vi "UHR-Fleezers Control (host) - 10.2.vi"() -> ()   [LabVIEW 2009] (continued)
                n756 = Build Array (concatenate)(w3470, w3469, w3463) -> (w3468:dbl[])
              }
              frame #1 {
                w3484 = 0.0 ("f")
                w3481 = FALSE ("Save APD Data\nwith Trap Data")
                # "calibration"
                n757 = Boolean To (0,1)(Boolean=w3481) -> (0, 1=w3486:i16)
                n758 = To Double Precision Float(number=w3486) -> (double precision float=w3485:dbl)
                n759 = Build Array(w3485, w3484, w3484, w3484, w3484) -> (w3483:dbl[])
                n760 = Build Array(w3482, w3487, w3487, w3494, w3493, 1.0 ("t")) -> (w3491:dbl[])
                n761 = Build Array (concatenate)(w3491, w3490, w3483) -> (w3489:dbl[])
                "Calibrating Trap..." <- TRUE ("Calibrating...")
              }
              frame #2 {
                w3501 = 0.0 ("f")
                # "scan dir (x/y = 0/1)"
                # "cycles/step"
                # "n scans (f/b)"
                # "steps"
                # "freq. range"
                # "AOD raster scan"
                n762 = local read "Number of F/B Scans (AOD)"() -> (w3508:u16)
                n763 = local read "Cycles/step (AOD)"() -> (w3510:u64)
                n764 = local read "Scan Range (MHz)"() -> (w3513:dbl)
                n765 = local read "Scan steps (AOD)"() -> (w3512:u64)
                n766 = local read "Scan BD"() -> (w3520:bool)
                n767 = local read "Save ave N"() -> (w3525:dbl)
                n768 = Boolean To (0,1)(Boolean=w3520) -> (0, 1=w3519:i16)
                n769 = To Double Precision Float(number=w3508) -> (double precision float=w3507:dbl)
                n770 = To Double Precision Float(number=w3512) -> (double precision float=w3511:dbl)
                n771 = To Double Precision Float(number=w3510) -> (double precision float=w3509:dbl)
                n772 = To Double Precision Float(number=w3519) -> (double precision float=w3518:dbl)
                n773 = Multiply(x=w3525, y=w3503) -> (x*y=w3524:dbl)
                n774 = To Double Precision Float(number=w3496) -> (double precision float=w3502:dbl)
                n775 = Build Array(w3502, w3501, w3501, w3501, w3501) -> (w3499:dbl[])
                n776 = local read "N sets should be saved"() -> (w3505:dbl)
                n777 = Build Array(w3518, w3513, w3511, w3509, w3507) -> (w3515:dbl[])
                n778 = Build Array(w3498, w3503, w3524, w3523, w3522, 2.0 ("t")) -> (w3517:dbl[])
                n779 = Round Toward +Infinity(x=w3505) -> (ceil(x): smallest int >= x=w3506:dbl)
                n780 = Build Array (concatenate)(w3517, w3516, w3499, w3515) -> (w3514:dbl[])
                n781 = To Unsigned Long Integer(number=w3506) -> (unsigned 32bit integer=w3504:u32)
              }
              frame #3 {
                w3534 = 0.0 ("f")
                # "MCL raster scan"
                n782 = local read "Number of scans (MCL)"() -> (w3529:u64)
                n783 = local read "Scan lines (y)"() -> (w3528:u64)
                n784 = local read "2D or 1D Scan"() -> (w3531:bool)
                n785 = local read "Scan Range (V)\n(of steps)"() -> (w3550:dbl)
                n786 = local read "Fast Scan Dir"() -> (w3557:bool)
                n787 = local read "Cycles/step (MCL)"() -> (w3547:u64)
                n788 = local read "Scan steps (MCL)"() -> (w3549:u64)
                n789 = Select(t=w3528, s=w3531, f=w3529) -> (s? t:f=w3530:u64)
                n790 = Boolean To (0,1)(Boolean=w3531) -> (0, 1=w3533:i16)
                n791 = local read "Save ave N"() -> (w3562:dbl)
                n792 = local read "Initial X"() -> (w3536:dbl)
                n793 = local read "Initial Y"() -> (w3535:dbl)
                n794 = To Double Precision Float(number=w3533) -> (double precision float=w3532:dbl)
                n795 = Boolean To (0,1)(Boolean=w3557) -> (0, 1=w3556:i16)
                n796 = To Double Precision Float(number=w3530) -> (double precision float=w3545:dbl)
                n797 = To Double Precision Float(number=w3549) -> (double precision float=w3548:dbl)
                n798 = To Double Precision Float(number=w3547) -> (double precision float=w3546:dbl)
                n799 = To Double Precision Float(number=w3556) -> (double precision float=w3555:dbl)
                n800 = Multiply(x=w3562, y=w3541) -> (x*y=w3561:dbl)
                n801 = To Double Precision Float(number=w3526) -> (double precision float=w3540:dbl)
                n802 = local read "N sets should be saved (MCL)"() -> (w3543:dbl)
                n803 = Build Array(w3540, w3532, w3534, w3534, w3534) -> (w3538:dbl[])
                n804 = Build Array(w3555, w3550, w3548, w3546, w3545, w3536, w3535) -> (w3552:dbl[])
                n805 = Build Array(w3537, w3541, w3561, w3560, w3559, 3.0 ("t")) -> (w3554:dbl[])
                n806 = Round Toward +Infinity(x=w3543) -> (ceil(x): smallest int >= x=w3544:dbl)
                n807 = Build Array (concatenate)(w3554, w3553, w3538, w3552) -> (w3551:dbl[])
                n808 = To Unsigned Long Integer(number=w3544) -> (unsigned 32bit integer=w3542:u32)
              }
            }
            n809 = local read "Index"() -> (w3401:dbl)
            n810 = call "Create new save file.vi"("Insert"="", "Ext"=".dat", "Index In"=w3401) -> ("Path Out"=w3360:path, "Index Out"=w3373:dbl)
            n811 = local write "Save file name"(w3360) -> ()
            n812 = local write "Index"(w3373) -> ()
            n813 = local write "Save index"(w3373) -> ()
            n814 = Array Size(array=w3384) -> (size(s)=w3385:i32)
            n815 = Open/Create/Replace File(file path (use dialog)=w3360, operation (0:open)=T33."create", access (0:read/write)=enum16{"read/write", "read-only", "write-only"}."write-only") -> (refnum out=w3398:refnum<file>)  [unwired: 1 in, 4 out]
            n816 = local write "Saving..."(TRUE ("Saving...")) -> ()
            n817 = To Double Precision Float(number=w3385) -> (double precision float=w3383:dbl)
            n818 = String Length(string="Comment (data description)") -> (length=w3381:i32)
            n819 = To Double Precision Float(number=w3381) -> (double precision float=w3380:dbl)
            n820 = Deny Access(7:w3398) -> (3:w3397:refnum<file>)  [unwired: 1 in, 2 out]
            n821 = Build Array (concatenate)(w3383, w3384, w3380) -> (w3382:dbl[])
            n822 = case shown="True" w3358 {
              tunnel: w3360 -> [_ w3412]
              tunnel: [refnum<k0> refnum w3411] -> w3359
              frame #0 {
              }
              frame #1 {
                w3407 = 0.0 ("element")
                n823 = Path To String(path=w3412) -> (string=w3426:string)
                n824 = Build Array(w3407, w3407, w3407, w3407, w3407, w3407, w3407, w3407) -> (w3408:dbl[])
                n825 = String Length(string=w3426) -> (length=w3425:i32)
                n826 = Subtract(x=w3425, y=4) -> (x-y=w3423:i32)
                n827 = Array Size(array=w3408) -> (size(s)=w3410:i32)
                n828 = String Subset(string=w3426, length (rest)=w3423) -> (substring=w3422:string)  [unwired: 1 out]
                n829 = To Double Precision Float(number=w3410) -> (double precision float=w3409:dbl)
                n830 = Concatenate Strings(w3422, "_pos.dat" ("string")) -> (w3420:string)
                n831 = Build Array (concatenate)(w3409, w3408) -> (w3406:dbl[])
                n832 = String To Path(string=w3420) -> (path=w3416:path)
                n833 = Open/Create/Replace File(file path (use dialog)=w3416, operation (0:open)=T33."create", access (0:read/write)=enum16{"read/write", "read-only", "write-only"}."write-only") -> (refnum out=w3417:refnum<file>)  [unwired: 1 in, 4 out]
                n834 = Deny Access(7:w3417) -> (3:w3413:refnum<file>)  [unwired: 1 in, 2 out]
                n835 = Write to Binary File(file (use dialog)=w3413, data=w3406, 5:FALSE ("prepend array or string size? (T)"), 9:T34."big-endian, network order" ("byte order (0:big-endian, network order)")) -> (refnum out=w3411:refnum<file>)  [unwired: 1 in, 3 out]
              }
            }
            n836 = case "If fluorescence data to be saved" shown="True" w3371 {
              tunnel: w3360 -> [_ w3450]
              tunnel: [refnum<k0> refnum w3430] -> w3372
              frame #0 {
              }
              frame #1 {
                w3429 = 0.0
                n837 = local read "APD Integration Time (s)"() -> (w3435:dbl)
                n838 = local read "N APD Samp/step"() -> (w3428:dbl)
                n839 = Path To String(path=w3450) -> (string=w3449:string)
                n840 = String Length(string=w3449) -> (length=w3448:i32)
                n841 = Subtract(x=w3448, y=4) -> (x-y=w3446:i32)
                n842 = String Subset(string=w3449, length (rest)=w3446) -> (substring=w3445:string)  [unwired: 1 out]
                n843 = Build Array(w3435, w3428, w3429, w3429, w3429, w3429, w3429, w3429) -> (w3432:dbl[])
                n844 = Concatenate Strings(w3445, "_fl.dat" ("string")) -> (w3443:string)
                n845 = Array Size(array=w3432) -> (size(s)=w3434:i32)
                n846 = String To Path(string=w3443) -> (path=w3439:path)
                n847 = Open/Create/Replace File(file path (use dialog)=w3439, operation (0:open)=T33."create", access (0:read/write)=enum16{"read/write", "read-only", "write-only"}."write-only") -> (refnum out=w3440:refnum<file>)  [unwired: 1 in, 4 out]
                n848 = Deny Access(7:w3440) -> (3:w3436:refnum<file>)  [unwired: 1 in, 2 out]
                n849 = To Double Precision Float(number=w3434) -> (double precision float=w3433:dbl)
                n850 = Build Array (concatenate)(w3433, w3432) -> (w3431:dbl[])
                n851 = Write to Binary File(file (use dialog)=w3436, data=w3431, 5:FALSE ("prepend array or string size? (T)"), 9:T34."big-endian, network order" ("byte order (0:big-endian, network order)")) -> (refnum out=w3430:refnum<file>)  [unwired: 1 in, 3 out]
              }
            }
            n852 = Write to Binary File(file (use dialog)=w3397, data=w3382, 5:w3378, 9:w3376) -> (refnum out=w3379:refnum<file>)  [unwired: 1 in, 3 out]
            n853 = Write to Binary File(file (use dialog)=w3379, data="Comment (data description)", 5:w3378, 9:w3376) -> (refnum out=w3375:refnum<file>)  [unwired: 1 in, 3 out]
          }
        }
      }
      frame #1 {
        n854 = local read "Saving..."() -> (w3575:bool)
        n855 = case shown="True" w3575 {
          tunnel: w3579 -> [_ w3589]
          tunnel: w3578 -> [_ w3603]
          tunnel: w3577 -> [_ w3599]
          tunnel: w3576 -> [_ w3598]
          tunnel: w3574 -> [_ w3597]
          tunnel: w3573 -> [_ w3592]
          tunnel: w3572 -> [_ w3591]
          tunnel: w3571 -> [_ w3590]
          tunnel: w3570 -> [_ w3588]
          tunnel: w3569 -> [_ w3586]
          tunnel: w3568 -> [_ w3585]
          tunnel: w3567 -> [_ w3584]
          tunnel: w3566 -> [_ w3583]
          tunnel: w3565 -> [_ w3582]
          tunnel: w3564 -> [_ w3581]
          tunnel: w3563 -> [_ w3580]
          frame #0 {
          }
          frame #1 {
            n856 = Multiply(x=w3589, y=w3588) -> (x*y=→"Time (s)":dbl)
            n857 = Less Or Equal?(x=w3589, y=w3597) -> (x <= y?=w3601:bool)
            n858 = Or(x="Stop Saving", y="Abort save 2") -> (x .or. y?=w3593:bool)
            n859 = Not(x=w3593) -> (.not. x?=w3602:bool)
            n860 = And(x=w3601, y=w3602) -> (x .and. y?=w3600:bool)
            n861 = case shown="True" w3600 {
              tunnel: w3603 -> [w3610 w3678]
              tunnel: [0.0 w3681] -> w3596
              tunnel: w3589 -> [_ w3679]
              tunnel: w3597 -> [_ w3680]
              tunnel: w3599 -> [_ w3675]
              tunnel: w3598 -> [_ _]
              tunnel: w3592 -> [w3608 w3668]
              tunnel: w3591 -> [w3607 w3669]
              tunnel: w3590 -> [_ w3667]
              tunnel: w3586 -> [_ w3666]
              tunnel: w3585 -> [_ w3620]
              tunnel: w3584 -> [_ w3659]
              tunnel: w3583 -> [_ w3637]
              tunnel: w3582 -> [w3604 w3618]
              tunnel: w3581 -> [w3605 w3617]
              tunnel: w3580 -> [_ w3614]
              frame #0 {
                w3606 = FALSE
                n862 = Close File(refnum=w3610) -> ()  [unwired: 1 in, 2 out]
                n863 = case shown="True" w3607 {
                  tunnel: w3608 -> [_ w3612]
                  frame #0 {
                  }
                  frame #1 {
                    n864 = Close File(refnum=w3612) -> ()  [unwired: 1 in, 2 out]
                  }
                }
                n865 = case shown="True" w3604 {
                  tunnel: w3605 -> [_ w3611]
                  frame #0 {
                  }
                  frame #1 {
                    n866 = Close File(refnum=w3611) -> ()  [unwired: 1 in, 2 out]
                  }
                }
                n867 = local write "Raster Scanning..."(w3606) -> ()
                n868 = local write "Calibrating Trap..."(w3606) -> ()
                n869 = call <vilib>:"Beep.vi"() -> ()  [unwired: 3 in, 9 out]
                n870 = local write "Stop Saving"(w3606) -> ()
                "Saving..." <- w3606
              }
              frame #1 {
                n871 = local read "Calibrating Trap..."() -> (w3670:bool)
                n872 = case "Write fl. data" shown="True" w3669 {
                  tunnel: w3668 -> [_ w3704]
                  tunnel: w3667 -> [_ w3703]
                  frame #0 {
                  }
                  frame #1 {
                    n873 = Write to Binary File(file (use dialog)=w3704, data=w3703, 5:FALSE ("prepend array or string size? (T)"), 9:T34."big-endian, network order" ("byte order (0:big-endian, network order)")) -> ()  [unwired: 1 in, 4 out]
                  }
                }
                n874 = Greater?(x="Save ave N", y=1.0) -> (0:w3673:bool)
                n875 = Not(x=w3670) -> (.not. x?=w3672:bool)
                n876 = And(x=w3672, y=w3673) -> (x .and. y?=w3615:bool)
                n877 = case shown="True" w3615 {
                  tunnel: w3614 -> [w3684 w3695]
                  tunnel: [w3684 w3687] -> w3613
                  tunnel: "Save ave N" -> [_ w3688]
                  frame #0 {
                  }
                  frame #1 {
                    w3685 = 2 ("dimension size")
                    n878 = Array Size(array=w3695) -> (size(s)=w3689:i32)
                    n879 = Divide(x=w3689, y=w3685) -> (x/y=w3693:dbl)
                    n880 = Reshape Array(w3695, w3693, w3685) -> (w3694:u64[][])
                    n881 = Transpose 2D Array(2D array=w3694) -> (transposed array=w3692:u64[][])
                    n882 = for {
                      tunnel: w3692 -> [w3697] mode=indexing
                      tunnel: [w3696] -> w3686 mode=indexing
                      tunnel: w3688 -> [w3698]
                      workers-P: _ -> [_]
                      n883 = call "downsample 1D array - U64.vi"("Ave N"=w3698, "Array In"=w3697) -> ("Array Out"=w3696:u64[])  [unwired: 1 in]
                    }
                    n884 = Transpose 2D Array(2D array=w3686) -> (transposed array=w3691:u64[][])
                    n885 = Divide(x=w3689, y=w3688) -> (x/y=w3690:dbl)
                    n886 = Reshape Array(w3691, w3690) -> (w3687:u64[])
                  }
                }
                n887 = case shown="True" w3615 {
                  tunnel: w3675 -> [w3707 w3719]
                  tunnel: [w3707 w3711] -> w3671
                  tunnel: "Save ave N" -> [_ w3712]
                  tunnel: w3666 -> [_ w3710]
                  frame #0 {
                  }
                  frame #1 {
                    n888 = Array Size(array=w3719) -> (size(s)=w3713:i32)
                    n889 = Array Size(array=w3710) -> (size(s)=w3709:i32)
                    n890 = Divide(x=w3713, y=w3709) -> (x/y=w3717:dbl)
                    n891 = Reshape Array(w3719, w3717, w3709) -> (w3718:i16[][])
                    n892 = Transpose 2D Array(2D array=w3718) -> (transposed array=w3716:i16[][])
                    n893 = for {
                      tunnel: w3716 -> [w3722] mode=indexing
                      tunnel: [w3721] -> w3708 mode=indexing
                      tunnel: w3712 -> [w3720]
                      workers-P: _ -> [_]
                      n894 = call "downsample 1D array - I16.vi"("Ave N"=w3720, "Array In"=w3722) -> ("Array Out"=w3721:i16[])  [unwired: 1 out]
                    }
                    n895 = Transpose 2D Array(2D array=w3708) -> (transposed array=w3715:i16[][])
                    n896 = Divide(x=w3713, y=w3712) -> (x/y=w3714:dbl)
                    n897 = Reshape Array(w3715, w3714) -> (w3711:i16[])
                  }
                }
                n898 = Index Array(array=w3637, index=1) -> (element=w3640:waveform(dbl))
                n899 = Index Array(array=w3637, index=0) -> (element=w3642:waveform(dbl))
                n900 = Unbundle By Name(w3640) -> ("Y"=w3644:dbl[])
                n901 = Unbundle By Name(w3642) -> ("Y"=w3652:dbl[])
                n902 = case "Write trap pos. data" shown="True" w3618 {
                  tunnel: w3617 -> [_ w3700]
                  tunnel: w3613 -> [_ w3699]
                  frame #0 {
                  }
                  frame #1 {
                    n903 = Write to Binary File(file (use dialog)=w3700, data=w3699, 5:FALSE ("prepend array or string size? (T)"), 9:T34."big-endian, network order" ("byte order (0:big-endian, network order)")) -> ()  [unwired: 1 in, 4 out]
                  }
                }
                n904 = Write to Binary File(file (use dialog)=w3678, data=w3671, 5:FALSE ("prepend array or string size? (T)"), 9:T34."big-endian, network order" ("byte order (0:big-endian, network order)")) -> ()  [unwired: 1 in, 4 out]
                n905 = feedback #26(w3644) -> (w3646:dbl[])
                n906 = Build Array (concatenate)(w3646, w3644) -> (w3645:dbl[])
                n907 = Select(t=w3644, s=w3620, f=w3645) -> (s? t:f=w3630:dbl[])
                n908 = feedback #27(w3652) -> (w3665:dbl[])
                n909 = Build Array (concatenate)(w3665, w3652) -> (w3664:dbl[])
                n910 = Select(t=w3652, s=w3620, f=w3664) -> (s? t:f=w3639:dbl[])
                n911 = Divide(x=w3679, y=w3680) -> (x/y=w3682:dbl)
                n912 = Multiply(x=w3682, y=100.0) -> (x*y=w3681:dbl)
                n913 = Build Array(w3639, w3630) -> (→"Saved APD":dbl[][])
                n914 = Array Size(array=w3639) -> (size(s)=w3657:i32)
                n915 = Unbundle By Name(w3659) -> ("Y"=w3663:dbl[])
                n916 = Subtract(x=w3657, y="N pts to average") -> (x-y=w3633:i32)
                n917 = Multiply(x="N pts to average", y=u16 2) -> (x*y=w3634:u16)
                n918 = Subtract(x=w3657, y=w3634) -> (x-y=w3632:i32)
                n919 = feedback #28(w3663) -> (w3662:dbl[])
                n920 = Build Array (concatenate)(w3662, w3663) -> (w3661:dbl[])
                n921 = Select(t=w3663, s=w3620, f=w3661) -> (s? t:f=w3660:dbl[])
                "Trap Delta Graph" <- w3660
                n922 = Array Subset(array=w3639, index=w3633, length="N pts to average") -> (w3656:dbl[])
                n923 = Array Subset(array=w3639, index=w3632, length="N pts to average") -> (w3655:dbl[])
                n924 = Array Subset(array=w3630, index=w3633, length="N pts to average") -> (w3636:dbl[])
                n925 = Array Subset(array=w3630, index=w3632, length="N pts to average") -> (w3635:dbl[])
                n926 = call <vilib>:"Mean.vi"("X"=w3656) -> ("mean"=w3654:dbl)  [unwired: 1 out]
                n927 = call <vilib>:"Mean.vi"("X"=w3636) -> ("mean"=w3629:dbl)  [unwired: 1 out]
                n928 = call <vilib>:"Mean.vi"("X"=w3655) -> ("mean"=w3653:dbl)  [unwired: 1 out]
                n929 = call <vilib>:"Mean.vi"("X"=w3635) -> ("mean"=w3628:dbl)  [unwired: 1 out]
                n930 = Subtract(x=w3629, y=w3628) -> (x-y=w3619:dbl)
                "Delta Fl. 2" <- w3619
                n931 = Subtract(x=w3654, y=w3653) -> (x-y=w3651:dbl)
                "Delta Fl. 1" <- w3651
                n932 = Initialize Array(w3651, 1 ("dimension size")) -> (w3648:dbl[])
                n933 = Initialize Array(w3619, 1 ("dimension size")) -> (w3625:dbl[])
                n934 = feedback #29(w3648) -> (w3649:dbl[])
                n935 = Build Array (concatenate)(w3649, w3648) -> (w3647:dbl[])
                n936 = feedback #30(w3625) -> (w3626:dbl[])
                n937 = Build Array (concatenate)(w3626, w3625) -> (w3624:dbl[])
                n938 = Select(t=w3648, s=w3620, f=w3647) -> (s? t:f=w3623:dbl[])
                n939 = Select(t=w3625, s=w3620, f=w3624) -> (s? t:f=w3622:dbl[])
                n940 = Build Array(w3623, w3622) -> (→"Save APD Deriv":dbl[][])
              }
            }
            "Progress" <- w3596
            "Progress 2" <- w3596
          }
        }
      }
    }
    n941 = Bundle By Name(cluster=w927, "Green FB Ch 0"=w926, "Green FB Ch 1"=w925) -> (w905:T41)
    "Green FB Signals (V)" <- w905
    n942 = Unbundle By Name(w905) -> ("Green FB Ch 2"=→"Green FB Plot":dbl)
    n943 = local read "wait to reset values"() -> (w997:bool)
    n944 = Not(x=w994) -> (.not. x?=w998:bool)
    n945 = And(x=w998, y=w997) -> (x .and. y?=w999:bool)
    n946 = case "Part of MCL raster scanning: returns to initial positions after scan done" shown="True" w999 {
      tunnel: w1002 -> [w2371 w2378]
      tunnel: [w2371 w2377] -> w1001
      tunnel: w996 -> [w2370 w2376]
      tunnel: [w2370 w2375] -> w995
      frame #0 {
      }
      frame #1 {
        w2386 = 10.0 ("y")
        w2385 = 32767.0 ("y")
        # "to return scan values\nafter a synchronous \nAOM scan"
        n947 = local read "AO2"() -> (w2379:dbl)
        n948 = local read "AO1"() -> (w2380:dbl)
        n949 = Multiply(x=w2380, y=w2385) -> (x*y=w2382:dbl)
        n950 = local write "wait to reset values"(FALSE ("wait to reset values")) -> ()
        n951 = Multiply(x=w2379, y=w2385) -> (x*y=w2384:dbl)
        n952 = Divide(x=w2382, y=w2386) -> (x/y=w2381:dbl)
        n953 = Divide(x=w2384, y=w2386) -> (x/y=w2383:dbl)
        n954 = To Word Integer(number=w2381) -> (16bit integer=w2387:i16)
        n955 = To Word Integer(number=w2383) -> (16bit integer=w2388:i16)
        n956 = local read "Total Counts (ticks)"() -> (w2372:u32)
        n957 = xnode "Read/Write Control"("FPGA VI Reference In"=w2378, "error in"=w2376, "AO1"=w2387, "AO2"=w2388, "MCL count"=w2372) -> ("FPGA VI Reference Out"=w2377:T21, "error out"=w2375:errorcluster)
        n958 = local read "Scan Range (V)\n(of steps)"() -> (w2373:dbl)
        n959 = property on="Scan Range (V)\n(of steps)" class="DigNum (strict)"("Val(Sgnl)"=w2373) -> ()  [unwired: 2 in, 2 out]
      }
    }
    n960 = node-c288() -> ()  [unwired: 2 out]
  }
  n961 = disable-structure shown="Disabled" {
    disable-tunnel: [w3796 _] -> w205
    disable-tunnel: w8 -> [w3795 _]
    frame #0 {
      n962 = node-c288() -> (w3798:T23)  [unwired: 4 out]
      n963 = timed-loop "Rough control of MCL mirror stage (debugging)" {
        tunnel: w3795 -> [w3801]
        tunnel: [w3800] -> w3796
        timing: w3798 -> [_]
        timing-out: [_] -> w3797
        stop <- w3800 stop-if-true
        n964 = node-c288() -> ()  [unwired: 2 out]
        n965 = case shown="1" "MCL Mode" {
          tunnel: w3801 -> [_ w3804 w3906]
          frame #0 {
          }
          frame #1 {
            n966 = node-c288() -> (w3806:T23)  [unwired: 4 out]
            n967 = timed-loop "Oscillate MCL mirror" {
              timing: w3806 -> [_]
              timing-out: [_] -> w3805
              tunnel: w3804 -> [w3845]
              i -> [w3844]
              stop <- w3807 stop-if-true
              n968 = node-c288() -> (w3843:i64)  [unwired: 1 out]
              n969 = Multiply(x="AO1", y=32767.0) -> (x*y=w3839:dbl)
              n970 = Multiply(x="AO2", y=32767.0) -> (x*y=w3834:dbl)
              n971 = Divide(x=w3839, y=10.0) -> (x/y=w3840:dbl)
              n972 = Divide(x=w3834, y=10.0) -> (x/y=w3835:dbl)
              n973 = To Word Integer(number=w3840) -> (16bit integer=w3832:i16)
              n974 = To Word Integer(number=w3835) -> (16bit integer=w3831:i16)
              n975 = Divide(x=w3843, y=i64 1000) -> (x/y=w3814:dbl)
              n976 = Multiply(x=w3814, y=w3844) -> (x*y=w3825:dbl)
              n977 = Multiply(x="Osc. freq. (Hz) 2", y=6.283185307179586) -> (x*y=w3826:dbl)
              n978 = Multiply(x=w3826, y=w3825) -> (x*y=w3824:dbl)
              n979 = Sine(x=w3824) -> (sin(x)=w3823:dbl)
              n980 = Multiply(x=w3823, y="Osc. amp. (V)") -> (x*y=w3821:dbl)
              n981 = Add(x=w3821, y="Osc. center (V)") -> (x+y=w3819:dbl)
              n982 = Divide(x=w3819, y=10.0) -> (x/y=w3817:dbl)
              n983 = Multiply(x=w3817, y=32767.0) -> (x*y=w3812:dbl)
              n984 = Select(t=w3812, s="Scan axis", f=w3832) -> (s? t:f=w3830:dbl)
              n985 = Select(t=w3831, s="Scan axis", f=w3812) -> (s? t:f=w3829:dbl)
              n986 = local read "MCL Mode"() -> (w3811:u16)
              n987 = Not Equal?(x=w3811, y=u16 1) -> (x != y?=w3808:bool)
              n988 = local read "Stop All"() -> (w3809:bool)
              n989 = xnode "Read/Write Control"("FPGA VI Reference In"=w3845, "AO1"=w3830, "AO2"=w3829) -> ()  [unwired: 1 in, 2 out]
              n990 = Compound Arithmetic op=OR(w3809, w3808) -> (w3807:bool)
              n991 = node-c288() -> ()  [unwired: 2 out]
            }
            n992 = node-c288(w3805) -> ()  [unwired: 1 out]
          }
          frame #2 {
            n993 = case shown="True" "Start Scan" {
              tunnel: w3906 -> [_ w3918]
              frame #0 {
              }
              frame #1 {
                n994 = Subtract(x="End (V)", y="Begin (V)") -> (x-y=w3914:dbl)
                n995 = Decrement(x="N Points") -> (x-1=w3913:dbl)
                n996 = Divide(x=w3914, y=w3913) -> (x/y=w3911:dbl)
                n997 = for {
                  N: "N Points" -> [_]
                  tunnel: "Begin (V)" -> [w3931]
                  tunnel: w3918 -> [w3923]
                  tunnel: [w3922] -> w3917 mode=indexing
                  tunnel: w3911 -> [w3921]
                  tunnel: [w3919] -> w3910 mode=indexing
                  i -> [w3930]
                  n998 = Multiply(x=w3921, y=w3930) -> (x*y=w3929:dbl)
                  n999 = Add(x=w3931, y=w3929) -> (x+y=w3926:dbl)
                  n1000 = local read "Scan axis"() -> (w3920:bool)
                  n1001 = local read "AO1"() -> (w3928:dbl)
                  n1002 = local read "AO2"() -> (w3927:dbl)
                  n1003 = Select(t=w3926, s=w3920, f=w3928) -> (s? t:f=w3925:dbl)
                  n1004 = Select(t=w3927, s=w3920, f=w3926) -> (s? t:f=w3924:dbl)
                  n1005 = flat-sequence {
                    tunnel: w3925 -> [w3935]
                    tunnel: w3924 -> [w3934]
                    tunnel: w3923 -> [w3932]
                    tunnel: [w4000] -> w3922
                    tunnel: [w3999] -> w3919
                    frame #0 {
                      w3938 = 10.0 ("y")
                      w3933 = 32767.0 ("y")
                      n1006 = Multiply(x=w3935, y=w3933) -> (x*y=w3941:dbl)
                      n1007 = Multiply(x=w3934, y=w3933) -> (x*y=w3939:dbl)
                      n1008 = Divide(x=w3941, y=w3938) -> (x/y=w3942:dbl)
                      n1009 = Divide(x=w3939, y=w3938) -> (x/y=w3940:dbl)
                      n1010 = To Word Integer(number=w3942) -> (16bit integer=w3936:i16)
                      n1011 = To Word Integer(number=w3940) -> (16bit integer=w3937:i16)
                      n1012 = xnode "Read/Write Control"("FPGA VI Reference In"=w3932, "AO1"=w3936, "AO2"=w3937) -> ()  [unwired: 1 in, 2 out]
                    }
                    frame #1 {
                      n1013 = Wait (ms)(milliseconds to wait="DAQ Delay (ms)") -> ()  [unwired: 1 out]
                    }
                    frame #2 {
                      n1014 = local read "Slow mean"() -> (w4000:dbl)
                      n1015 = local read "Sigma"() -> (w3999:dbl)
                    }
                  }
                }
                n1016 = Bundle("Begin (V)"="Begin (V)", w3911, w3917) -> (→"MCL Scan":cluster{"Begin (V)":dbl, dbl, dbl[]})  [unwired: 1 out]
                n1017 = Bundle("Begin (V)"="Begin (V)", w3911, w3910) -> (→"MCL Scan 2":cluster{"Begin (V)":dbl, dbl, dbl[]})  [unwired: 1 out]
              }
            }
          }
        }
        n1018 = local read "Stop All"() -> (w3800:bool)
        n1019 = node-c288() -> ()  [unwired: 2 out]
      }
      n1020 = node-c288(w3797) -> ()  [unwired: 1 out]
    }
    frame #1 {
    }
  }
  n1021 = timed-loop "Control parameters (event loop)" {
    tunnel: w8 -> [w4007]
    shift-right: [w4006] -> _
    shift-left: errorcluster {"status"=FALSE, "code"=0, "source"=""} ("error out") -> [w4005]
    tunnel: [w4004] -> w203
    timing: w50 -> [_]
    timing-out: [_] -> w49
    tunnel: w22 -> [w4003]
    stop <- w4004 stop-if-true
    n1022 = node-c288() -> ()  [unwired: 2 out]
    n1023 = event shown="[43] \"Sample Channel Flow\": Value Change" {
      selector: _ -> [_ _ _ _ _ _ _ _ _ _ _ _ _ _ _ _ _ _ _ _ _ _ _ _ _ _ _ _ _ _ _ _ _ _ _ _ _ _ _ _ _ _ _ _ _ _ _ _ _ _ _ _ _]
      dyn-events: _ -> [_ _ _ _ _ _ _ _ _ _ _ _ _ _ _ _ _ _ _ _ _ _ _ _ _ _ _ _ _ _ _ _ _ _ _ _ _ _ _ _ _ _ _ _ _ _ _ _ _ _ _ _ _]
      timeout: _ -> [_ _ _ _ _ _ _ _ _ _ _ _ _ _ _ _ _ _ _ _ _ _ _ _ _ _ _ _ _ _ _ _ _ _ _ _ _ _ _ _ _ _ _ _ _ _ _ _ _ _ _ _ _]
      tunnel: w4007 -> [w4045 _ _ _ w4164 _ w4259 _ _ _ _ w4325 _ _ w4425 w4563 w4625 w4668 w4818 w4893 w5004 w5097 w5181 w5265 w5349 w5433 w5517 w5608 w5765 w5971 w6064 w6197 _ w6367 w6408 w6455 w6532 w6573 _ w6618 _ _ _ _ w6799 _ w6890 w6930 w6976 w7112 w7161 _ w7221]
      tunnel: [w4044 _ _ _ w4154 _ w4258 _ _ w4290 _ w4304 _ _ w4424 w4559 w4622 w4665 w4817 w4891 w5003 w5091 w5175 w5259 w5343 w5427 w5511 w5606 w5764 w5969 w6062 w6195 _ w6365 w6406 w6445 w6530 w6571 _ w6616 _ _ _ _ w6797 _ _ _ _ _ _ _ _] -> w4006
      tunnel: w4005 -> [w4043 _ _ _ w4163 _ w4257 _ _ w4290 _ w4324 _ _ w4423 w4558 w4621 w4664 w4816 w4892 w5002 w5096 w5180 w5264 w5348 w5432 w5516 w5607 w5763 w5970 w6063 w6196 _ w6366 w6407 w6454 w6531 w6572 _ w6617 _ _ _ _ w6798 _ w6889 w6929 w6975 w7111 w7160 _ w7220]
      tunnel: [_ _ _ _ _ _ _ _ _ w4289 _ _ _ _ _ _ _ _ _ _ _ _ _ _ _ _ _ _ _ _ _ _ _ _ _ _ _ _ _ _ _ _ _ _ _ _ _ _ _ _ _ _ _] -> w4004
      tunnel: [_ _ _ _ _ _ _ "Round T1 X" _ _ _ _ _ _ _ _ _ _ _ _ _ _ _ _ _ _ _ _ _ _ _ _ _ _ _ _ _ _ _ _ _ _ _ _ _ _ _ _ _ _ _ _ _] -> _
      tunnel: [_ _ _ "Adjust Scale\nto Mean" _ _ _ _ _ _ _ _ _ _ _ _ _ _ _ _ _ _ _ _ _ _ _ _ _ _ _ _ _ _ _ _ _ _ _ _ _ _ _ _ _ _ _ _ _ _ _ _ _] -> _
      tunnel: [_ _ _ _ _ _ _ _ "Round T2 X" _ "Delayed Interlace Start" _ _ _ _ _ _ _ _ _ _ _ _ _ _ _ _ _ _ _ _ _ _ _ _ _ _ _ _ _ _ _ _ _ _ _ _ _ _ _ _ _ _] -> _
      tunnel: w4003 -> [_ _ _ _ _ _ _ _ _ _ _ _ _ _ _ _ _ _ _ _ _ _ _ _ _ _ _ _ _ _ _ _ _ _ _ _ _ _ _ _ _ _ _ w6790 _ _ _ _ _ _ _ _ _]
      event #0 {
        # "So that if 'Save ave N' is updated, the AOD scanning code updates too."
        n1024 = event-data() -> ()  [unwired: 6 out]
        n1025 = local read "AI Count (ticks)"() -> (w4025:u32)
        n1026 = Boolean To (0,1)(Boolean="Sets to FIFO (Traps)") -> (0, 1=w4035:cluster{"Set 1":i16, "Set 2":i16, "Set 3":i16})
        n1027 = xnode "Read/Write Control"("FPGA VI Reference In"=w4045, "error in"=w4043, "ai count"=w4025, "AI1 Sets to FIFO"="Sets to FIFO (Traps)", "N of AI1 Int Acq Sets"="N Acq Sets (Traps + Fl.)") -> ("error out"=w4044:errorcluster)  [unwired: 1 out]
        n1028 = Cluster To Array(cluster=w4035) -> (array=w4034:i16[])
        n1029 = To Unsigned Long Integer(number=w4034) -> (unsigned 32bit integer=w4014:u32[])
        n1030 = local read "Scan steps (AOD)"() -> (w4036:u64)
        n1031 = Multiply(x=w4025, y="N Acq Sets (Traps + Fl.)") -> (x*y=w4023:u32)
        n1032 = Divide(x=40000000.0, y=w4025) -> (x/y=w4017:dbl)
        "AI rate (Hz)" <- w4017
        "Ave. Rate (Hz)" <- w4017
        n1033 = Add Array Elements(numeric array=w4014) -> (sum=w4026:u32)
        "Trap Sets" <- w4026
        n1034 = Reciprocal(x=w4017) -> (1/x=→"Ave. Period (s)":dbl)
        n1035 = property on="Scan steps (AOD)" class="DigNum (strict)"("Val(Sgnl)"=w4036) -> ()  [unwired: 2 in, 2 out]
        n1036 = Divide(x=w4017, y="N Acq Sets (Traps + Fl.)") -> (x/y=w4040:dbl)
        "Data Rate (Hz)" <- w4040
        n1037 = Reciprocal(x=w4040) -> (1/x=→"Data Period (s)":dbl)
        n1038 = local read "Save ave N"() -> (w4039:dbl)
        n1039 = Divide(x=w4040, y=w4039) -> (x/y=w4038:dbl)
        "Save Data Rate (Hz)" <- w4038
        n1040 = Reciprocal(x=w4038) -> (1/x=→"Save Data Period (s)":dbl)
        n1041 = Multiply(x=w4023, y="# Samples/trap") -> (x*y=w4021:u32)
        "Counts/DMA" <- w4021
        n1042 = property on="Trap Disp. Downsample" class="DigNum (strict)"("Maximum"="# Samples/trap") -> ()  [unwired: 2 in, 2 out]
        n1043 = Multiply(x=w4026, y="# Samples/trap") -> (x*y=w4015:u32)
        "# Samples/channel" <- w4015
        n1044 = Multiply(x=w4015, y=u32 8) -> (x*y=→"Trap AI Elements/DMA read":u32)
        n1045 = local read "APD Int. Count"() -> (w4022:u32)
        n1046 = Multiply(x=w4015, y=u32 3) -> (x*y=→"Trap Pos Elements/DMA read":u32)
        n1047 = Divide(x=w4021, y=w4022) -> (x/y=w4012:dbl)
        "APD Samples/FIFO Acq." <- w4012
        n1048 = Divide(x=w4021, y=40000000.0) -> (x/y=w4019:dbl)
        "DMA Update Period (s)" <- w4019
        n1049 = Multiply(x=2.0, y=w4012) -> (x*y=→"APD Elements/DMA read":dbl)
        n1050 = property on="APD Disp. Downsample" class="DigNum (strict)"("Maximum"=w4012) -> ()  [unwired: 2 in, 2 out]
        n1051 = local read "N sets to save"() -> (w4032:u32)
        n1052 = Multiply(x=w4019, y=w4032) -> (x*y=→"Total Time (s)":dbl)
        "FPGA Averaging" <- FALSE ("FPGA Averaging")
      }
      event #1 {
        n1053 = event-data() -> ()  [unwired: 7 out]
        n1054 = And(x=FALSE, y="Rescale on Mean") -> (x .and. y?=w4129:bool)
        n1055 = local write "Rescale on Mean"(w4129) -> ()
        n1056 = local read "Bead Mean (nm)"() -> (w4134:dbl)
        n1057 = Add(x="Amplitude (nm)", y=w4134) -> (x+y=w4132:dbl)
        n1058 = Subtract(x=w4134, y="Amplitude (nm)") -> (x-y=w4131:dbl)
        n1059 = property on="Bead Separation" class="WFChart (strict)"("YScale.Minimum"=w4131) -> ()  [unwired: 2 in, 2 out]
        n1060 = property on="Bead Separation" class="WFChart (strict)"("YScale.Maximum"=w4132) -> ()  [unwired: 2 in, 2 out]
      }
      event #2 {
        n1061 = event-data() -> ()  [unwired: 7 out]
        n1062 = local read "AI labels"() -> (w4135:string[])
        n1063 = property on="High Res. Display" class="Ring (strict)"("Strings []"=w4135) -> ()  [unwired: 2 in, 2 out]
        n1064 = Build Array (concatenate)(w4135, "none") -> (w4136:string[])
        n1065 = property on="FFT 1 Choice 1" class="Ring (strict)"("Strings []"=w4136) -> ()  [unwired: 2 in, 2 out]
        n1066 = property on="FFT 1 Choice 2" class="Ring (strict)"("Strings []"=w4136) -> ()  [unwired: 2 in, 2 out]
        n1067 = property on="FFT 2 Choice 1" class="Ring (strict)"("Strings []"=w4136) -> ()  [unwired: 2 in, 2 out]
        n1068 = property on="FFT 2 Choice 2" class="Ring (strict)"("Strings []"=w4136) -> ()  [unwired: 2 in, 2 out]
        n1069 = Bundle("APD 1", "APD 2") -> (w4139:cluster{string, string})  [unwired: 1 out]
        n1070 = Cluster To Array(cluster=w4139) -> (array=w4137:string[])
        n1071 = Build Array (concatenate)(w4137, w4136) -> (w4141:string[])
        n1072 = Array Size(array=w4141) -> (size(s)=w4142:i32)
        n1073 = property on="Signals to Plot" class="LstBox (strict)"("Item Names"=w4141) -> ()  [unwired: 2 in, 2 out]
        n1074 = property on="Signals to Plot" class="LstBox (strict)"("Number of Rows"=w4142) -> ()  [unwired: 2 in, 2 out]
        n1075 = property on="All Signals" class="WFChart (strict)"("LegNumRows"=w4142) -> ()  [unwired: 2 in, 2 out]
      }
      event #3 {
        n1076 = event-data() -> ()  [unwired: 7 out]
        n1077 = local read "APD 1 Rate (Hz)"() -> (w4151:dbl)
        n1078 = Multiply(x=1000.0, y="Above (kHz)") -> (x*y=w4149:dbl)
        n1079 = Multiply(x=1000.0, y="Below (kHz)") -> (x*y=w4147:dbl)
        n1080 = Add(x=w4149, y=w4151) -> (x+y=w4144:dbl)
        n1081 = Subtract(x=w4151, y=w4147) -> (x-y=w4145:dbl)
        n1082 = property on="APD Chart" class="WFChart (strict)"("YScale.Minimum"=w4145) -> ()  [unwired: 2 in, 2 out]
        n1083 = property on="APD Chart" class="WFChart (strict)"("YScale.Maximum"=w4144) -> ()  [unwired: 2 in, 2 out]
      }
      event #4 {
        n1084 = event-data() -> ()  [unwired: 7 out]
        n1085 = Negate(x="Phase adj. (AI1)") -> (-x=w4161:i16)
        n1086 = Select(t=w4161, s="- phase (AI1)", f="Phase adj. (AI1)") -> (s? t:f=w4160:i16)
        n1087 = xnode "Read/Write Control"("FPGA VI Reference In"=w4164, "error in"=w4163, "Phase count adjustment"=w4160) -> ("FPGA VI Reference Out"=w4159:T21, "error out"=w4158:errorcluster)
        n1088 = Or(x="- phase (AI1)", y="+ phase (AI1)") -> (x .or. y?=w4155:bool)
        n1089 = xnode "Read/Write Control"("FPGA VI Reference In"=w4159, "error in"=w4158, "+ phase"=w4155) -> ("error out"=w4154:errorcluster)  [unwired: 1 out]
      }
      event #5 {
        w4240 = u32 9868950 ("Color Box")
        n1090 = event-data() -> ("Row"=w4242:i32)  [unwired: 9 out]
        n1091 = property on="All Signals" class="WFChart (strict)"("Active Plot"=w4242) -> (error out=w4253:errorcluster)  [unwired: 2 in, 1 out]
        n1092 = property on="All Signals" class="WFChart (strict)" props=["Plot", "Visible?", "Plot", "Plot Color"](error in=w4253) -> (error out=w4252:errorcluster, "Plot.Visible?"=w4251:bool)  [unwired: 1 in, 2 out]
        n1093 = Select(t=FALSE ("Plot.Visible"), s=w4251, f=TRUE ("Plot.Visible")) -> (s? t:f=w4246:bool)
        n1094 = property on="All Signals" class="WFChart (strict)"(error in=w4252, "Plot.Visible?"=w4246) -> (error out=w4248:errorcluster)  [unwired: 1 in, 1 out]
        n1095 = property on="All Signals" class="WFChart (strict)"(error in=w4248) -> (error out=w4243:errorcluster, "Plot.Plot Color"=w4247:u32)  [unwired: 1 in, 1 out]
        n1096 = property on="Signals to Plot" class="LstBox (strict)"(error in=w4243, "Active Row"=w4242) -> (error out=w4241:errorcluster)  [unwired: 1 in, 1 out]
        n1097 = Select(t=w4247, s=w4246, f=u32 0) -> (s? t:f=w4244:u32)
        n1098 = property on="Signals to Plot" class="LstBox (strict)"(error in=w4241, "CellFontColor"=w4244, "SelColor"=w4240, "CellBG"=w4240, "CellFontSize"=u32 20 ("Active Row:Cell Font:Size"), "CellFontBold"=TRUE ("Active Row:Cell Font:Bold")) -> ()  [unwired: 1 in, 2 out]
      }
      event #6 {
        n1099 = event-data() -> ("CtlRef"=w4256:refnum<vi>)  [unwired: 6 out]
        n1100 = control-ref of="Trap Delta (MHz)"() -> (w4255:refnum<vi>)
        n1101 = Equal?(x=w4255, y=w4256) -> (x = y?=w4254:bool)
        n1102 = case shown="False" "Oscillate Set 1" {
          tunnel: w4259 -> [w4279 _]
          tunnel: [w4278 w4282] -> w4258
          tunnel: w4257 -> [w4277 w4282]
          tunnel: w4254 -> [w4262 _]
          frame #0 {
            n1103 = local read "BD 1 Frequency 2 (MHz)"() -> (w4266:dbl)
            n1104 = local read "BD 1 Frequency 1 (MHz)"() -> (w4264:dbl)
            n1105 = Subtract(x=w4266, y="Trap Delta (MHz)") -> (x-y=w4263:dbl)
            n1106 = Select(t=w4263, s=w4262, f=w4264) -> (s? t:f=w4261:dbl)
            n1107 = local read "Y RF Frequency Limits (MHz)"() -> (w4267:T16)
            n1108 = local read "X RF Frequency Limits (MHz)"() -> (w4268:T16)
            n1109 = local read "BD 1 Frequency 3 (MHz)"() -> (w4280:dbl)
            n1110 = local write "BD 1 Frequency 1 (MHz)"(w4261) -> ()
            n1111 = local read "BD 2 Frequency 1 (MHz)"() -> (w4271:dbl)
            n1112 = local read "BD 2 Frequency 2 (MHz)"() -> (w4270:dbl)
            n1113 = local read "BD 2 Frequency 3 (MHz)"() -> (w4281:dbl)
            n1114 = call "set RF board frequency - interlace.vi"("Board 2 Frequency Limits"=w4267, "Board 1 Frequency Limits"=w4268, "error in"=w4277, "FPGA VI Reference In"=w4279, "Board 2 Frequency 3 (MHz)"=w4281, "Board 1 Frequency 3 (MHz)"=w4280, "Board 2 Frequency 2 (MHz)"=w4270, "Board 2 Frequency 1 (MHz)"=w4271, "Board 1 Frequency 2 (MHz)"=w4266, "Board 1 Frequency 1  (MHz)"=w4261) -> ("error out"=w4278:errorcluster)  [unwired: 1 out]
            n1115 = Subtract(x=w4271, y=w4270) -> (x-y=w4275:dbl)
            n1116 = Subtract(x=w4261, y=w4266) -> (x-y=w4276:dbl)
            n1117 = Square(x=w4275) -> (x^2=w4273:dbl)
            n1118 = Square(x=w4276) -> (x^2=w4274:dbl)
            n1119 = Add(x=w4274, y=w4273) -> (x+y=w4272:dbl)
            n1120 = Square Root(x=w4272) -> (sqrt(x)=w4269:dbl)
            n1121 = local write "Trap Delta (MHz)"(w4269) -> ()
            n1122 = property on="Initial delta (MHz)" class="DigNum (strict)"("Val(Sgnl)"=w4269) -> ()  [unwired: 2 in, 2 out]
          }
          frame #1 {
          }
        }
      }
      event #7 {
        n1123 = event-data() -> ()  [unwired: 7 out]
        n1124 = local read "BD 1 Frequency 1 (MHz)"() -> (w4285:dbl)
        n1125 = Round To Nearest(number=w4285) -> (nearest integer value=w4284:dbl)
        n1126 = property on="BD 1 Frequency 1 (MHz)" class="DigNum (strict)"("Val(Sgnl)"=w4284) -> ()  [unwired: 2 in, 2 out]
      }
      event #8 {
        n1127 = event-data() -> ()  [unwired: 7 out]
        n1128 = local read "BD 1 Frequency 2 (MHz)"() -> (w4287:dbl)
        n1129 = Round To Nearest(number=w4287) -> (nearest integer value=w4286:dbl)
        n1130 = property on="BD 1 Frequency 2 (MHz)" class="DigNum (strict)"("Val(Sgnl)"=w4286) -> ()  [unwired: 2 in, 2 out]
      }
      event #9 {
        n1131 = event-data() -> ()  [unwired: 7 out]
        n1132 = local read "Stop All"() -> (w4289:bool)
      }
      event #10 {
        n1133 = event-data() -> ()  [unwired: 7 out]
        n1134 = flat-sequence {
          frame #0 {
            n1135 = Multiply(x="Delay to Interlace (s)", y=1000.0) -> (x*y=w4292:dbl)
            n1136 = Wait (ms)(milliseconds to wait=w4292) -> ()  [unwired: 1 out]
          }
          frame #1 {
            n1137 = property on="Green laser mode" class="RadioBtnsControl (strict)"("Val(Sgnl)"=enum32{"Laser ON", "Laser OFF", "Interlace"}."Interlace" ("Value (Signaling)")) -> ()  [unwired: 2 in, 2 out]
          }
        }
      }
      event #11 {
        w4316 = i16 1 ("f")
        n1138 = event-data() -> ()  [unwired: 7 out]
        n1139 = local write "Trap 1 (ON/OFF)"("Trap 1 ON") -> ()
        n1140 = local write "Trap 2 (ON/OFF)"("Trap 2 ON") -> ()
        n1141 = Boolean To (0,1)(Boolean="Trap 3 ON") -> (0, 1=w4317:i16)
        n1142 = Boolean To (0,1)(Boolean="Trap 1 ON") -> (0, 1=w4318:i16)
        n1143 = Boolean To (0,1)(Boolean="Trap 2 ON") -> (0, 1=w4319:i16)
        n1144 = Select(t=w4319, s="Trap ON/OFF X or Y Amp?", f=w4316) -> (s? t:f=w4314:i16)
        n1145 = Select(t=w4318, s="Trap ON/OFF X or Y Amp?", f=w4316) -> (s? t:f=w4315:i16)
        n1146 = Select(t=w4317, s="Trap ON/OFF X or Y Amp?", f=w4316) -> (s? t:f=w4313:i16)
        n1147 = Select(t=w4316, s="Trap ON/OFF X or Y Amp?", f=w4319) -> (s? t:f=w4311:i16)
        n1148 = Select(t=w4316, s="Trap ON/OFF X or Y Amp?", f=w4318) -> (s? t:f=w4312:i16)
        n1149 = Select(t=w4316, s="Trap ON/OFF X or Y Amp?", f=w4317) -> (s? t:f=w4310:i16)
        n1150 = And(x="All FB On/Off", y="Feedback On/Off") -> (x .and. y?=w4308:cluster{"Set 1":bool, "Set 2":bool})
        n1151 = local read "BD 1 Amplitude 1 (%)"() -> (w4328:dbl)
        n1152 = local read "BD 1 Amplitude 2 (%)"() -> (w4327:dbl)
        n1153 = local read "BD 1 Amplitude 3 (%)"() -> (w4326:dbl)
        n1154 = Unbundle By Name(w4308) -> ("Set 1"=w4303:bool, "Set 2"=w4300:bool)
        n1155 = local read "Y RF Amplitude Limits (%)"() -> (w4296:T16)
        n1156 = local read "X RF Amplitude Limits (%)"() -> (w4297:T16)
        n1157 = local read "BD 2 Amplitude 1 (%)"() -> (w4329:dbl)
        n1158 = local read "BD 2 Amplitude 2 (%)"() -> (w4330:dbl)
        n1159 = local read "BD 2 Amplitude 3 (%)"() -> (w4331:dbl)
        n1160 = And(x="Trap 2 ON", y=w4300) -> (x .and. y?=w4298:bool)
        n1161 = And(x="Trap 1 ON", y=w4303) -> (x .and. y?=w4301:bool)
        n1162 = Multiply(x=w4315, y=w4328) -> (x*y=w4323:dbl)
        n1163 = Multiply(x=w4327, y=w4314) -> (x*y=w4321:dbl)
        n1164 = Multiply(x=w4326, y=w4313) -> (x*y=w4322:dbl)
        n1165 = Multiply(x=w4329, y=w4312) -> (x*y=w4332:dbl)
        n1166 = Multiply(x=w4330, y=w4311) -> (x*y=w4333:dbl)
        n1167 = Multiply(x=w4331, y=w4310) -> (x*y=w4334:dbl)
        n1168 = call "set RF board amplitude - interlace.vi"("Board 2 Amplitude Limits"=w4296, "Board 1 Amplitude Limits"=w4297, "error in"=w4324, "FPGA VI Reference In"=w4325, "Board 2 Amplitude 3 (%)"=w4334, "Board 1 Amplitude 3 (%)"=w4322, "Board 2 Amplitude 2 (%)"=w4333, "Board 2 Amplitude 1 (%)"=w4332, "Board 1 Amplitude 2 (%)"=w4321, "Board 1 Amplitude 1 (%)"=w4323) -> ("error out"=w4305:errorcluster, "FPGA VI Reference Out"=w4306:T21)
        n1169 = xnode "Read/Write Control"("FPGA VI Reference In"=w4306, "error in"=w4305, "FB On/Off Set 1"=w4301, "FB On/Off Set 2"=w4298) -> ("error out"=w4304:errorcluster)  [unwired: 1 out]
      }
      event #12 {
        n1170 = event-data() -> ()  [unwired: 7 out]
        n1171 = property on="Saved AOD Raster Scan Parameter Sets" class="Arr (strict)"() -> ("Index Values"=w4402:u32[])  [unwired: 2 in, 2 out]
        n1172 = Index Array(array=w4402, index=0) -> (element=w4399:u32)
        n1173 = local write "Load parameters"(FALSE ("Load parameters")) -> ()
        n1174 = Index Array(array="Saved AOD Raster Scan Parameter Sets", index=w4399) -> (element=w4398:T42)
        n1175 = Unbundle By Name(w4398) -> ("Scan Range AOD (nm) 2"=w4397:dbl, "Step Size AOD (nm) 2"=w4396:dbl, "Scan Speed AOD (nm/s) 2"=w4395:dbl, "Number of scans (AOD) 2"=w4394:u16)
        n1176 = flat-sequence {
          tunnel: w4397 -> [w4405]
          tunnel: w4396 -> [w4404]
          tunnel: w4395 -> [w4403]
          tunnel: w4394 -> [w4406]
          frame #0 {
            n1177 = local write "Scan Speed (nm/s)"(w4403) -> ()
            n1178 = local write "Scan Range (nm)"(w4405) -> ()
            n1179 = local write "Step Size (nm)"(w4404) -> ()
          }
          frame #1 {
            n1180 = property on="Number of F/B Scans (AOD)" class="DigNum (strict)"("Val(Sgnl)"=w4406) -> ()  [unwired: 2 in, 2 out]
          }
        }
      }
      event #13 {
        n1181 = event-data() -> ()  [unwired: 7 out]
        n1182 = property on="Trap 2 ON" class="Bool (strict)"("Val(Sgnl)"="Trap 2 (ON/OFF)") -> ()  [unwired: 2 in, 2 out]
        n1183 = property on="Trap 1 ON" class="Bool (strict)"("Val(Sgnl)"="Trap 1 (ON/OFF)") -> ()  [unwired: 2 in, 2 out]
      }
      event #14 {
        n1184 = event-data() -> ()  [unwired: 7 out]
        n1185 = local read "DIO count 3 (ticks)"() -> (w4419:u32)
        n1186 = local read "DIO count 1 (ticks)"() -> (w4421:u32)
        n1187 = local read "DIO count 2 (ticks)"() -> (w4420:u32)
        n1188 = To Unsigned Byte Integer(number="Not-Interlacing Set") -> (unsigned 8bit integer=w4410:u8)
        n1189 = Add(x=w4410, y=u8 1) -> (x+y=w4414:u8)
        n1190 = xnode "Read/Write Control"("FPGA VI Reference In"=w4425, "error in"=w4423, "DIO count 1 (ticks)"=w4421, "DIO count 2 (ticks)"=w4420, "DIO count 3 (ticks)"=w4419, "Interlace ON/OFF"="Interlace", "Number Interlace Cycles"="Number Interlace Sets", "Interlace Off Parameters"=w4414) -> ("error out"=w4424:errorcluster)  [unwired: 1 out]
        n1191 = Build Array(w4421, w4420, w4419) -> (w4412:u32[])
        n1192 = Split 1D Array(array=w4412, index="Number Interlace Sets") -> (first subarray=w4422:u32[])  [unwired: 1 out]
        n1193 = Index Array(array=w4412, index=w4410) -> (element=w4411:u32)
        n1194 = Add Array Elements(numeric array=w4422) -> (sum=w4416:u32)
        n1195 = Select(t=w4416, s="Interlace", f=w4411) -> (s? t:f=→"Total Counts (ticks)":u32)
      }
      event #15 {
        n1196 = event-data() -> ()  [unwired: 7 out]
        n1197 = Unbundle By Name("Reset Feedback") -> ("Set 1"=w4561:bool, "Set 2"=w4560:bool)
        n1198 = xnode "Read/Write Control"("FPGA VI Reference In"=w4563, "error in"=w4558, "FB Reset Set 1"=w4561, "FB Reset Set 2"=w4560) -> ("error out"=w4559:errorcluster)  [unwired: 1 out]
      }
      event #16 {
        n1199 = event-data() -> ()  [unwired: 7 out]
        n1200 = Unbundle By Name("PID Gains") -> ("Set 1"=w4624:T14, "Set 2"=w4623:T14)
        n1201 = xnode "Read/Write Control"("FPGA VI Reference In"=w4625, "error in"=w4621, "FB Gains Set 1"=w4624, "FB Gains Set 2"=w4623) -> ("error out"=w4622:errorcluster)  [unwired: 1 out]
      }
      event #17 {
        n1202 = event-data() -> ()  [unwired: 7 out]
        n1203 = xnode "Read/Write Control"("FPGA VI Reference In"=w4668, "error in"=w4664) -> ("FPGA VI Reference Out"=w4667:T21, "error out"=w4666:errorcluster, "AI2 Y Sum Set 1"=w4675:i16, "AI2 Y Sum Set 2"=w4674:i16)
        n1204 = Cluster To Array(cluster="AI2 to Setpoint") -> (array=w4678:bool[])